vi "1D history all datatypes.vi"   [LabVIEW 2021, in "Ring Buffer Strict Accessor Unit Tests.lvlib"]
uses:
  Ring Buffer Strict Accessor Unit Tests.lvlib
  ffb6f79c-0e8b-4f28-b3ed-bf3963fddc00.vi
  dcb4b22f-e317-4554-9adc-d9d904393cee.vi
  860586e6-507f-4244-af87-8e25528c7787.vi
  04da1d12-4007-43e6-bd40-3bc5b4287603.vi
  d3cdd860-2221-4504-b2d7-d7ebb0f0ee59.vi
  ecb8fbaa-c9af-4774-8849-7f352d3a9ee1.vi
  dba9704d-e78e-47f3-8626-fce484395582.vi
  112621f5-6873-4c6d-a91b-c9d1466c59a4.vi
  7b287e7a-98f1-404d-bc95-c25095b4fc31.vi
  fa233392-5b64-4c8c-836f-c43556db6967.vi
  6d70e3f0-6966-4327-968b-3c5b2aebe7d0.vi
  ffb6f79c-0e8b-4f28-b3ed-bf3963fddc00.vi/8499afdd-f86a-4785-a8f1-e7a09133571a.vi
  ffb6f79c-0e8b-4f28-b3ed-bf3963fddc00.vi/38752bf6-7fea-4fd6-9295-87f253133584.vi
  ffb6f79c-0e8b-4f28-b3ed-bf3963fddc00.vi/d2d864d0-4a0d-406a-953d-2a5df2a8b7c4.vi
  ffb6f79c-0e8b-4f28-b3ed-bf3963fddc00.vi/8f65235b-2f25-4f49-b818-5875480b4ea3.vi
  dcb4b22f-e317-4554-9adc-d9d904393cee.vi/8499afdd-f86a-4785-a8f1-e7a09133571a.vi
  dcb4b22f-e317-4554-9adc-d9d904393cee.vi/38752bf6-7fea-4fd6-9295-87f253133584.vi
  dcb4b22f-e317-4554-9adc-d9d904393cee.vi/d2d864d0-4a0d-406a-953d-2a5df2a8b7c4.vi
  dcb4b22f-e317-4554-9adc-d9d904393cee.vi/8f65235b-2f25-4f49-b818-5875480b4ea3.vi
  860586e6-507f-4244-af87-8e25528c7787.vi/8499afdd-f86a-4785-a8f1-e7a09133571a.vi
  860586e6-507f-4244-af87-8e25528c7787.vi/38752bf6-7fea-4fd6-9295-87f253133584.vi
  860586e6-507f-4244-af87-8e25528c7787.vi/d2d864d0-4a0d-406a-953d-2a5df2a8b7c4.vi
  860586e6-507f-4244-af87-8e25528c7787.vi/8f65235b-2f25-4f49-b818-5875480b4ea3.vi
  04da1d12-4007-43e6-bd40-3bc5b4287603.vi/8499afdd-f86a-4785-a8f1-e7a09133571a.vi
  04da1d12-4007-43e6-bd40-3bc5b4287603.vi/38752bf6-7fea-4fd6-9295-87f253133584.vi
  04da1d12-4007-43e6-bd40-3bc5b4287603.vi/d2d864d0-4a0d-406a-953d-2a5df2a8b7c4.vi
  04da1d12-4007-43e6-bd40-3bc5b4287603.vi/8f65235b-2f25-4f49-b818-5875480b4ea3.vi
  d3cdd860-2221-4504-b2d7-d7ebb0f0ee59.vi/8499afdd-f86a-4785-a8f1-e7a09133571a.vi
  d3cdd860-2221-4504-b2d7-d7ebb0f0ee59.vi/38752bf6-7fea-4fd6-9295-87f253133584.vi
  d3cdd860-2221-4504-b2d7-d7ebb0f0ee59.vi/d2d864d0-4a0d-406a-953d-2a5df2a8b7c4.vi
  d3cdd860-2221-4504-b2d7-d7ebb0f0ee59.vi/8f65235b-2f25-4f49-b818-5875480b4ea3.vi
  ecb8fbaa-c9af-4774-8849-7f352d3a9ee1.vi/8499afdd-f86a-4785-a8f1-e7a09133571a.vi
  ecb8fbaa-c9af-4774-8849-7f352d3a9ee1.vi/38752bf6-7fea-4fd6-9295-87f253133584.vi
  ecb8fbaa-c9af-4774-8849-7f352d3a9ee1.vi/d2d864d0-4a0d-406a-953d-2a5df2a8b7c4.vi
  ecb8fbaa-c9af-4774-8849-7f352d3a9ee1.vi/8f65235b-2f25-4f49-b818-5875480b4ea3.vi
  dba9704d-e78e-47f3-8626-fce484395582.vi/8499afdd-f86a-4785-a8f1-e7a09133571a.vi
  dba9704d-e78e-47f3-8626-fce484395582.vi/38752bf6-7fea-4fd6-9295-87f253133584.vi
  dba9704d-e78e-47f3-8626-fce484395582.vi/d2d864d0-4a0d-406a-953d-2a5df2a8b7c4.vi
  dba9704d-e78e-47f3-8626-fce484395582.vi/8f65235b-2f25-4f49-b818-5875480b4ea3.vi
  112621f5-6873-4c6d-a91b-c9d1466c59a4.vi/8499afdd-f86a-4785-a8f1-e7a09133571a.vi
  112621f5-6873-4c6d-a91b-c9d1466c59a4.vi/38752bf6-7fea-4fd6-9295-87f253133584.vi
  112621f5-6873-4c6d-a91b-c9d1466c59a4.vi/d2d864d0-4a0d-406a-953d-2a5df2a8b7c4.vi
  112621f5-6873-4c6d-a91b-c9d1466c59a4.vi/8f65235b-2f25-4f49-b818-5875480b4ea3.vi
  7b287e7a-98f1-404d-bc95-c25095b4fc31.vi/8499afdd-f86a-4785-a8f1-e7a09133571a.vi
  7b287e7a-98f1-404d-bc95-c25095b4fc31.vi/38752bf6-7fea-4fd6-9295-87f253133584.vi
  7b287e7a-98f1-404d-bc95-c25095b4fc31.vi/d2d864d0-4a0d-406a-953d-2a5df2a8b7c4.vi
  7b287e7a-98f1-404d-bc95-c25095b4fc31.vi/8f65235b-2f25-4f49-b818-5875480b4ea3.vi
  fa233392-5b64-4c8c-836f-c43556db6967.vi/8499afdd-f86a-4785-a8f1-e7a09133571a.vi
  fa233392-5b64-4c8c-836f-c43556db6967.vi/38752bf6-7fea-4fd6-9295-87f253133584.vi
  fa233392-5b64-4c8c-836f-c43556db6967.vi/d2d864d0-4a0d-406a-953d-2a5df2a8b7c4.vi
  fa233392-5b64-4c8c-836f-c43556db6967.vi/8f65235b-2f25-4f49-b818-5875480b4ea3.vi
  6d70e3f0-6966-4327-968b-3c5b2aebe7d0.vi/8499afdd-f86a-4785-a8f1-e7a09133571a.vi
  6d70e3f0-6966-4327-968b-3c5b2aebe7d0.vi/38752bf6-7fea-4fd6-9295-87f253133584.vi
  6d70e3f0-6966-4327-968b-3c5b2aebe7d0.vi/d2d864d0-4a0d-406a-953d-2a5df2a8b7c4.vi
  6d70e3f0-6966-4327-968b-3c5b2aebe7d0.vi/8f65235b-2f25-4f49-b818-5875480b4ea3.vi
  <userlib>/bjustice/Ring Buffer for Time Series Data/API Poly.vi
  <userlib>/bjustice/Ring Buffer for Time Series Data/API/Write Array.vi
  ffb6f79c-0e8b-4f28-b3ed-bf3963fddc00.vi/8499afdd-f86a-4785-a8f1-e7a09133571a.vi/f2df9050-0eef-46c6-aff6-3ce3a8893ea5.vi
  ffb6f79c-0e8b-4f28-b3ed-bf3963fddc00.vi/38752bf6-7fea-4fd6-9295-87f253133584.vi/17d75e1a-130a-47e0-8f2c-6c7d90b8ca77.vi
  <userlib>/bjustice/Ring Buffer for Time Series Data/API/Read Full Rotated Buffer.vi
  Source/SubVIs/Search for time to keep.vi
  Source/SubVIs/Index ByteArray.vi
  ffb6f79c-0e8b-4f28-b3ed-bf3963fddc00.vi/38752bf6-7fea-4fd6-9295-87f253133584.vi/19bdd28a-0674-4be3-87bb-ec701e431d75.vi
  Source/SubVIs/error if empty buffer.vi
  ffb6f79c-0e8b-4f28-b3ed-bf3963fddc00.vi/8f65235b-2f25-4f49-b818-5875480b4ea3.vi/4c2a6c61-f100-483c-8a49-51e57025a24c.vi
  ffb6f79c-0e8b-4f28-b3ed-bf3963fddc00.vi/8f65235b-2f25-4f49-b818-5875480b4ea3.vi/e57bc314-87c7-4952-9bc8-929005dac297.vi
  dcb4b22f-e317-4554-9adc-d9d904393cee.vi/8499afdd-f86a-4785-a8f1-e7a09133571a.vi/f2df9050-0eef-46c6-aff6-3ce3a8893ea5.vi
  dcb4b22f-e317-4554-9adc-d9d904393cee.vi/38752bf6-7fea-4fd6-9295-87f253133584.vi/17d75e1a-130a-47e0-8f2c-6c7d90b8ca77.vi
  dcb4b22f-e317-4554-9adc-d9d904393cee.vi/38752bf6-7fea-4fd6-9295-87f253133584.vi/19bdd28a-0674-4be3-87bb-ec701e431d75.vi
  dcb4b22f-e317-4554-9adc-d9d904393cee.vi/8f65235b-2f25-4f49-b818-5875480b4ea3.vi/4c2a6c61-f100-483c-8a49-51e57025a24c.vi
  dcb4b22f-e317-4554-9adc-d9d904393cee.vi/8f65235b-2f25-4f49-b818-5875480b4ea3.vi/e57bc314-87c7-4952-9bc8-929005dac297.vi
  860586e6-507f-4244-af87-8e25528c7787.vi/8499afdd-f86a-4785-a8f1-e7a09133571a.vi/f2df9050-0eef-46c6-aff6-3ce3a8893ea5.vi
  860586e6-507f-4244-af87-8e25528c7787.vi/38752bf6-7fea-4fd6-9295-87f253133584.vi/17d75e1a-130a-47e0-8f2c-6c7d90b8ca77.vi
  860586e6-507f-4244-af87-8e25528c7787.vi/38752bf6-7fea-4fd6-9295-87f253133584.vi/19bdd28a-0674-4be3-87bb-ec701e431d75.vi
  860586e6-507f-4244-af87-8e25528c7787.vi/8f65235b-2f25-4f49-b818-5875480b4ea3.vi/4c2a6c61-f100-483c-8a49-51e57025a24c.vi
  860586e6-507f-4244-af87-8e25528c7787.vi/8f65235b-2f25-4f49-b818-5875480b4ea3.vi/e57bc314-87c7-4952-9bc8-929005dac297.vi
  04da1d12-4007-43e6-bd40-3bc5b4287603.vi/8499afdd-f86a-4785-a8f1-e7a09133571a.vi/f2df9050-0eef-46c6-aff6-3ce3a8893ea5.vi
  04da1d12-4007-43e6-bd40-3bc5b4287603.vi/38752bf6-7fea-4fd6-9295-87f253133584.vi/17d75e1a-130a-47e0-8f2c-6c7d90b8ca77.vi
  04da1d12-4007-43e6-bd40-3bc5b4287603.vi/38752bf6-7fea-4fd6-9295-87f253133584.vi/19bdd28a-0674-4be3-87bb-ec701e431d75.vi
  04da1d12-4007-43e6-bd40-3bc5b4287603.vi/8f65235b-2f25-4f49-b818-5875480b4ea3.vi/4c2a6c61-f100-483c-8a49-51e57025a24c.vi
  04da1d12-4007-43e6-bd40-3bc5b4287603.vi/8f65235b-2f25-4f49-b818-5875480b4ea3.vi/e57bc314-87c7-4952-9bc8-929005dac297.vi
  d3cdd860-2221-4504-b2d7-d7ebb0f0ee59.vi/8499afdd-f86a-4785-a8f1-e7a09133571a.vi/f2df9050-0eef-46c6-aff6-3ce3a8893ea5.vi
  d3cdd860-2221-4504-b2d7-d7ebb0f0ee59.vi/38752bf6-7fea-4fd6-9295-87f253133584.vi/17d75e1a-130a-47e0-8f2c-6c7d90b8ca77.vi
  d3cdd860-2221-4504-b2d7-d7ebb0f0ee59.vi/38752bf6-7fea-4fd6-9295-87f253133584.vi/19bdd28a-0674-4be3-87bb-ec701e431d75.vi
  d3cdd860-2221-4504-b2d7-d7ebb0f0ee59.vi/8f65235b-2f25-4f49-b818-5875480b4ea3.vi/4c2a6c61-f100-483c-8a49-51e57025a24c.vi
  d3cdd860-2221-4504-b2d7-d7ebb0f0ee59.vi/8f65235b-2f25-4f49-b818-5875480b4ea3.vi/e57bc314-87c7-4952-9bc8-929005dac297.vi
  ecb8fbaa-c9af-4774-8849-7f352d3a9ee1.vi/8499afdd-f86a-4785-a8f1-e7a09133571a.vi/f2df9050-0eef-46c6-aff6-3ce3a8893ea5.vi
  ecb8fbaa-c9af-4774-8849-7f352d3a9ee1.vi/38752bf6-7fea-4fd6-9295-87f253133584.vi/17d75e1a-130a-47e0-8f2c-6c7d90b8ca77.vi
  ecb8fbaa-c9af-4774-8849-7f352d3a9ee1.vi/38752bf6-7fea-4fd6-9295-87f253133584.vi/19bdd28a-0674-4be3-87bb-ec701e431d75.vi
  ecb8fbaa-c9af-4774-8849-7f352d3a9ee1.vi/8f65235b-2f25-4f49-b818-5875480b4ea3.vi/4c2a6c61-f100-483c-8a49-51e57025a24c.vi
  ecb8fbaa-c9af-4774-8849-7f352d3a9ee1.vi/8f65235b-2f25-4f49-b818-5875480b4ea3.vi/e57bc314-87c7-4952-9bc8-929005dac297.vi
  dba9704d-e78e-47f3-8626-fce484395582.vi/8499afdd-f86a-4785-a8f1-e7a09133571a.vi/f2df9050-0eef-46c6-aff6-3ce3a8893ea5.vi
  dba9704d-e78e-47f3-8626-fce484395582.vi/38752bf6-7fea-4fd6-9295-87f253133584.vi/17d75e1a-130a-47e0-8f2c-6c7d90b8ca77.vi
  dba9704d-e78e-47f3-8626-fce484395582.vi/38752bf6-7fea-4fd6-9295-87f253133584.vi/19bdd28a-0674-4be3-87bb-ec701e431d75.vi
  dba9704d-e78e-47f3-8626-fce484395582.vi/8f65235b-2f25-4f49-b818-5875480b4ea3.vi/4c2a6c61-f100-483c-8a49-51e57025a24c.vi
  dba9704d-e78e-47f3-8626-fce484395582.vi/8f65235b-2f25-4f49-b818-5875480b4ea3.vi/e57bc314-87c7-4952-9bc8-929005dac297.vi
  112621f5-6873-4c6d-a91b-c9d1466c59a4.vi/8499afdd-f86a-4785-a8f1-e7a09133571a.vi/f2df9050-0eef-46c6-aff6-3ce3a8893ea5.vi
  112621f5-6873-4c6d-a91b-c9d1466c59a4.vi/38752bf6-7fea-4fd6-9295-87f253133584.vi/17d75e1a-130a-47e0-8f2c-6c7d90b8ca77.vi
  112621f5-6873-4c6d-a91b-c9d1466c59a4.vi/38752bf6-7fea-4fd6-9295-87f253133584.vi/19bdd28a-0674-4be3-87bb-ec701e431d75.vi
  112621f5-6873-4c6d-a91b-c9d1466c59a4.vi/8f65235b-2f25-4f49-b818-5875480b4ea3.vi/4c2a6c61-f100-483c-8a49-51e57025a24c.vi
  112621f5-6873-4c6d-a91b-c9d1466c59a4.vi/8f65235b-2f25-4f49-b818-5875480b4ea3.vi/e57bc314-87c7-4952-9bc8-929005dac297.vi
  7b287e7a-98f1-404d-bc95-c25095b4fc31.vi/8499afdd-f86a-4785-a8f1-e7a09133571a.vi/f2df9050-0eef-46c6-aff6-3ce3a8893ea5.vi
  7b287e7a-98f1-404d-bc95-c25095b4fc31.vi/38752bf6-7fea-4fd6-9295-87f253133584.vi/17d75e1a-130a-47e0-8f2c-6c7d90b8ca77.vi
  7b287e7a-98f1-404d-bc95-c25095b4fc31.vi/38752bf6-7fea-4fd6-9295-87f253133584.vi/19bdd28a-0674-4be3-87bb-ec701e431d75.vi
  7b287e7a-98f1-404d-bc95-c25095b4fc31.vi/8f65235b-2f25-4f49-b818-5875480b4ea3.vi/4c2a6c61-f100-483c-8a49-51e57025a24c.vi
  7b287e7a-98f1-404d-bc95-c25095b4fc31.vi/8f65235b-2f25-4f49-b818-5875480b4ea3.vi/e57bc314-87c7-4952-9bc8-929005dac297.vi
  fa233392-5b64-4c8c-836f-c43556db6967.vi/8499afdd-f86a-4785-a8f1-e7a09133571a.vi/f2df9050-0eef-46c6-aff6-3ce3a8893ea5.vi
  fa233392-5b64-4c8c-836f-c43556db6967.vi/38752bf6-7fea-4fd6-9295-87f253133584.vi/17d75e1a-130a-47e0-8f2c-6c7d90b8ca77.vi
  fa233392-5b64-4c8c-836f-c43556db6967.vi/38752bf6-7fea-4fd6-9295-87f253133584.vi/19bdd28a-0674-4be3-87bb-ec701e431d75.vi
  fa233392-5b64-4c8c-836f-c43556db6967.vi/8f65235b-2f25-4f49-b818-5875480b4ea3.vi/4c2a6c61-f100-483c-8a49-51e57025a24c.vi
  fa233392-5b64-4c8c-836f-c43556db6967.vi/8f65235b-2f25-4f49-b818-5875480b4ea3.vi/e57bc314-87c7-4952-9bc8-929005dac297.vi
  6d70e3f0-6966-4327-968b-3c5b2aebe7d0.vi/8499afdd-f86a-4785-a8f1-e7a09133571a.vi/f2df9050-0eef-46c6-aff6-3ce3a8893ea5.vi
  6d70e3f0-6966-4327-968b-3c5b2aebe7d0.vi/38752bf6-7fea-4fd6-9295-87f253133584.vi/17d75e1a-130a-47e0-8f2c-6c7d90b8ca77.vi
  6d70e3f0-6966-4327-968b-3c5b2aebe7d0.vi/38752bf6-7fea-4fd6-9295-87f253133584.vi/19bdd28a-0674-4be3-87bb-ec701e431d75.vi
  6d70e3f0-6966-4327-968b-3c5b2aebe7d0.vi/8f65235b-2f25-4f49-b818-5875480b4ea3.vi/4c2a6c61-f100-483c-8a49-51e57025a24c.vi
  6d70e3f0-6966-4327-968b-3c5b2aebe7d0.vi/8f65235b-2f25-4f49-b818-5875480b4ea3.vi/e57bc314-87c7-4952-9bc8-929005dac297.vi
  <userlib>/bjustice/Ring Buffer for Time Series Data/SubVIs/Split Values Array.vi
  <userlib>/bjustice/Ring Buffer for Time Series Data/SubVIs/Replace Values Array Multiple Timestamps.vi
  ffb6f79c-0e8b-4f28-b3ed-bf3963fddc00.vi/8499afdd-f86a-4785-a8f1-e7a09133571a.vi/f2df9050-0eef-46c6-aff6-3ce3a8893ea5.vi/63c583a5-c20f-4aba-9c90-661423dee4c4.vi
  ffb6f79c-0e8b-4f28-b3ed-bf3963fddc00.vi/8499afdd-f86a-4785-a8f1-e7a09133571a.vi/f2df9050-0eef-46c6-aff6-3ce3a8893ea5.vi/52385341-3d9c-45d2-aff5-e082a4793eb1.vi
  ffb6f79c-0e8b-4f28-b3ed-bf3963fddc00.vi/8499afdd-f86a-4785-a8f1-e7a09133571a.vi/f2df9050-0eef-46c6-aff6-3ce3a8893ea5.vi/37f29efa-f142-46b1-a185-f0098a95fbb6.vi
  ffb6f79c-0e8b-4f28-b3ed-bf3963fddc00.vi/8499afdd-f86a-4785-a8f1-e7a09133571a.vi/f2df9050-0eef-46c6-aff6-3ce3a8893ea5.vi/84b3d231-9afe-4b6e-afae-e0be43a31e4e.vi
  ffb6f79c-0e8b-4f28-b3ed-bf3963fddc00.vi/8499afdd-f86a-4785-a8f1-e7a09133571a.vi/f2df9050-0eef-46c6-aff6-3ce3a8893ea5.vi/c726271c-fc36-4bb7-8553-8945ec40c1cd.vi
  ffb6f79c-0e8b-4f28-b3ed-bf3963fddc00.vi/8499afdd-f86a-4785-a8f1-e7a09133571a.vi/f2df9050-0eef-46c6-aff6-3ce3a8893ea5.vi/a7b1d944-dc88-46f5-9d3e-305d46bbe1f6.vi
  ffb6f79c-0e8b-4f28-b3ed-bf3963fddc00.vi/8499afdd-f86a-4785-a8f1-e7a09133571a.vi/f2df9050-0eef-46c6-aff6-3ce3a8893ea5.vi/8abc4a6e-a1d2-4e85-879b-517e0ab55733.vi
  ffb6f79c-0e8b-4f28-b3ed-bf3963fddc00.vi/8499afdd-f86a-4785-a8f1-e7a09133571a.vi/f2df9050-0eef-46c6-aff6-3ce3a8893ea5.vi/bd347357-b475-4a03-9ac5-3b85ef11aecc.vi
  ffb6f79c-0e8b-4f28-b3ed-bf3963fddc00.vi/8499afdd-f86a-4785-a8f1-e7a09133571a.vi/f2df9050-0eef-46c6-aff6-3ce3a8893ea5.vi/391b36e9-a702-45e4-9499-3914f8833a58.vi
  ffb6f79c-0e8b-4f28-b3ed-bf3963fddc00.vi/8499afdd-f86a-4785-a8f1-e7a09133571a.vi/f2df9050-0eef-46c6-aff6-3ce3a8893ea5.vi/44155b33-c915-49ce-9e44-a66693aa70dd.vi
  ffb6f79c-0e8b-4f28-b3ed-bf3963fddc00.vi/8499afdd-f86a-4785-a8f1-e7a09133571a.vi/f2df9050-0eef-46c6-aff6-3ce3a8893ea5.vi/36977d53-dbe0-4dbc-b2ac-3dea4345b868.vi
  ffb6f79c-0e8b-4f28-b3ed-bf3963fddc00.vi/38752bf6-7fea-4fd6-9295-87f253133584.vi/17d75e1a-130a-47e0-8f2c-6c7d90b8ca77.vi/bbb64351-fa28-4ac1-b583-44e271193ecd.vi
  <userlib>/bjustice/Ring Buffer for Time Series Data/SubVIs/Rotate Buffer.vi
  Source/SubVIs/Search for oldest time to keep.vi
  Source/SubVIs/Search for newest time to keep.vi
  Source/SubVIs/datatype byte size.vi
  Source/SubVIs/array sizes to number of points.vi
  ffb6f79c-0e8b-4f28-b3ed-bf3963fddc00.vi/38752bf6-7fea-4fd6-9295-87f253133584.vi/19bdd28a-0674-4be3-87bb-ec701e431d75.vi/81c66277-30bd-484c-9c7c-9646f36721bb.vi
  ffb6f79c-0e8b-4f28-b3ed-bf3963fddc00.vi/38752bf6-7fea-4fd6-9295-87f253133584.vi/19bdd28a-0674-4be3-87bb-ec701e431d75.vi/7ca10173-70f1-4bfb-9c4b-948090662032.vi
  ffb6f79c-0e8b-4f28-b3ed-bf3963fddc00.vi/38752bf6-7fea-4fd6-9295-87f253133584.vi/19bdd28a-0674-4be3-87bb-ec701e431d75.vi/ea4aced9-3494-4b3f-b998-02af6afbdac4.vi
  ffb6f79c-0e8b-4f28-b3ed-bf3963fddc00.vi/38752bf6-7fea-4fd6-9295-87f253133584.vi/19bdd28a-0674-4be3-87bb-ec701e431d75.vi/022c581c-5349-49df-98f9-5a038829ee63.vi
  ffb6f79c-0e8b-4f28-b3ed-bf3963fddc00.vi/38752bf6-7fea-4fd6-9295-87f253133584.vi/19bdd28a-0674-4be3-87bb-ec701e431d75.vi/ed40bcc8-bbaa-4b61-9e1a-b4b75cf21b06.vi
  ffb6f79c-0e8b-4f28-b3ed-bf3963fddc00.vi/38752bf6-7fea-4fd6-9295-87f253133584.vi/19bdd28a-0674-4be3-87bb-ec701e431d75.vi/f4b703c2-aaab-40a0-b3da-b0c22dc82d50.vi
  ffb6f79c-0e8b-4f28-b3ed-bf3963fddc00.vi/38752bf6-7fea-4fd6-9295-87f253133584.vi/19bdd28a-0674-4be3-87bb-ec701e431d75.vi/1efa054f-b143-4d96-9f7e-584a7c6fa7fd.vi
  ffb6f79c-0e8b-4f28-b3ed-bf3963fddc00.vi/38752bf6-7fea-4fd6-9295-87f253133584.vi/19bdd28a-0674-4be3-87bb-ec701e431d75.vi/b7c29f3f-256a-4401-af9d-aa15374df391.vi
  ffb6f79c-0e8b-4f28-b3ed-bf3963fddc00.vi/38752bf6-7fea-4fd6-9295-87f253133584.vi/19bdd28a-0674-4be3-87bb-ec701e431d75.vi/2fb7b479-974d-4a18-8674-c4c8d9dc9a89.vi
  ffb6f79c-0e8b-4f28-b3ed-bf3963fddc00.vi/38752bf6-7fea-4fd6-9295-87f253133584.vi/19bdd28a-0674-4be3-87bb-ec701e431d75.vi/faac7175-5814-4bb6-a961-a8db1f460653.vi
  ffb6f79c-0e8b-4f28-b3ed-bf3963fddc00.vi/38752bf6-7fea-4fd6-9295-87f253133584.vi/19bdd28a-0674-4be3-87bb-ec701e431d75.vi/b6af2a6f-71a4-4cfe-837f-b196861458b0.vi
  dcb4b22f-e317-4554-9adc-d9d904393cee.vi/8499afdd-f86a-4785-a8f1-e7a09133571a.vi/f2df9050-0eef-46c6-aff6-3ce3a8893ea5.vi/63c583a5-c20f-4aba-9c90-661423dee4c4.vi
  dcb4b22f-e317-4554-9adc-d9d904393cee.vi/8499afdd-f86a-4785-a8f1-e7a09133571a.vi/f2df9050-0eef-46c6-aff6-3ce3a8893ea5.vi/52385341-3d9c-45d2-aff5-e082a4793eb1.vi
  dcb4b22f-e317-4554-9adc-d9d904393cee.vi/8499afdd-f86a-4785-a8f1-e7a09133571a.vi/f2df9050-0eef-46c6-aff6-3ce3a8893ea5.vi/37f29efa-f142-46b1-a185-f0098a95fbb6.vi
  dcb4b22f-e317-4554-9adc-d9d904393cee.vi/8499afdd-f86a-4785-a8f1-e7a09133571a.vi/f2df9050-0eef-46c6-aff6-3ce3a8893ea5.vi/84b3d231-9afe-4b6e-afae-e0be43a31e4e.vi
  dcb4b22f-e317-4554-9adc-d9d904393cee.vi/8499afdd-f86a-4785-a8f1-e7a09133571a.vi/f2df9050-0eef-46c6-aff6-3ce3a8893ea5.vi/c726271c-fc36-4bb7-8553-8945ec40c1cd.vi
  dcb4b22f-e317-4554-9adc-d9d904393cee.vi/8499afdd-f86a-4785-a8f1-e7a09133571a.vi/f2df9050-0eef-46c6-aff6-3ce3a8893ea5.vi/a7b1d944-dc88-46f5-9d3e-305d46bbe1f6.vi
  dcb4b22f-e317-4554-9adc-d9d904393cee.vi/8499afdd-f86a-4785-a8f1-e7a09133571a.vi/f2df9050-0eef-46c6-aff6-3ce3a8893ea5.vi/8abc4a6e-a1d2-4e85-879b-517e0ab55733.vi
  dcb4b22f-e317-4554-9adc-d9d904393cee.vi/8499afdd-f86a-4785-a8f1-e7a09133571a.vi/f2df9050-0eef-46c6-aff6-3ce3a8893ea5.vi/bd347357-b475-4a03-9ac5-3b85ef11aecc.vi
  dcb4b22f-e317-4554-9adc-d9d904393cee.vi/8499afdd-f86a-4785-a8f1-e7a09133571a.vi/f2df9050-0eef-46c6-aff6-3ce3a8893ea5.vi/391b36e9-a702-45e4-9499-3914f8833a58.vi
  dcb4b22f-e317-4554-9adc-d9d904393cee.vi/8499afdd-f86a-4785-a8f1-e7a09133571a.vi/f2df9050-0eef-46c6-aff6-3ce3a8893ea5.vi/44155b33-c915-49ce-9e44-a66693aa70dd.vi
  dcb4b22f-e317-4554-9adc-d9d904393cee.vi/8499afdd-f86a-4785-a8f1-e7a09133571a.vi/f2df9050-0eef-46c6-aff6-3ce3a8893ea5.vi/36977d53-dbe0-4dbc-b2ac-3dea4345b868.vi
  dcb4b22f-e317-4554-9adc-d9d904393cee.vi/38752bf6-7fea-4fd6-9295-87f253133584.vi/17d75e1a-130a-47e0-8f2c-6c7d90b8ca77.vi/bbb64351-fa28-4ac1-b583-44e271193ecd.vi
  dcb4b22f-e317-4554-9adc-d9d904393cee.vi/38752bf6-7fea-4fd6-9295-87f253133584.vi/19bdd28a-0674-4be3-87bb-ec701e431d75.vi/81c66277-30bd-484c-9c7c-9646f36721bb.vi
  dcb4b22f-e317-4554-9adc-d9d904393cee.vi/38752bf6-7fea-4fd6-9295-87f253133584.vi/19bdd28a-0674-4be3-87bb-ec701e431d75.vi/7ca10173-70f1-4bfb-9c4b-948090662032.vi
  dcb4b22f-e317-4554-9adc-d9d904393cee.vi/38752bf6-7fea-4fd6-9295-87f253133584.vi/19bdd28a-0674-4be3-87bb-ec701e431d75.vi/ea4aced9-3494-4b3f-b998-02af6afbdac4.vi
  dcb4b22f-e317-4554-9adc-d9d904393cee.vi/38752bf6-7fea-4fd6-9295-87f253133584.vi/19bdd28a-0674-4be3-87bb-ec701e431d75.vi/022c581c-5349-49df-98f9-5a038829ee63.vi
  dcb4b22f-e317-4554-9adc-d9d904393cee.vi/38752bf6-7fea-4fd6-9295-87f253133584.vi/19bdd28a-0674-4be3-87bb-ec701e431d75.vi/ed40bcc8-bbaa-4b61-9e1a-b4b75cf21b06.vi
  dcb4b22f-e317-4554-9adc-d9d904393cee.vi/38752bf6-7fea-4fd6-9295-87f253133584.vi/19bdd28a-0674-4be3-87bb-ec701e431d75.vi/f4b703c2-aaab-40a0-b3da-b0c22dc82d50.vi
  dcb4b22f-e317-4554-9adc-d9d904393cee.vi/38752bf6-7fea-4fd6-9295-87f253133584.vi/19bdd28a-0674-4be3-87bb-ec701e431d75.vi/1efa054f-b143-4d96-9f7e-584a7c6fa7fd.vi
  dcb4b22f-e317-4554-9adc-d9d904393cee.vi/38752bf6-7fea-4fd6-9295-87f253133584.vi/19bdd28a-0674-4be3-87bb-ec701e431d75.vi/b7c29f3f-256a-4401-af9d-aa15374df391.vi
  dcb4b22f-e317-4554-9adc-d9d904393cee.vi/38752bf6-7fea-4fd6-9295-87f253133584.vi/19bdd28a-0674-4be3-87bb-ec701e431d75.vi/2fb7b479-974d-4a18-8674-c4c8d9dc9a89.vi
  dcb4b22f-e317-4554-9adc-d9d904393cee.vi/38752bf6-7fea-4fd6-9295-87f253133584.vi/19bdd28a-0674-4be3-87bb-ec701e431d75.vi/faac7175-5814-4bb6-a961-a8db1f460653.vi
  dcb4b22f-e317-4554-9adc-d9d904393cee.vi/38752bf6-7fea-4fd6-9295-87f253133584.vi/19bdd28a-0674-4be3-87bb-ec701e431d75.vi/b6af2a6f-71a4-4cfe-837f-b196861458b0.vi
  860586e6-507f-4244-af87-8e25528c7787.vi/8499afdd-f86a-4785-a8f1-e7a09133571a.vi/f2df9050-0eef-46c6-aff6-3ce3a8893ea5.vi/63c583a5-c20f-4aba-9c90-661423dee4c4.vi
  860586e6-507f-4244-af87-8e25528c7787.vi/8499afdd-f86a-4785-a8f1-e7a09133571a.vi/f2df9050-0eef-46c6-aff6-3ce3a8893ea5.vi/52385341-3d9c-45d2-aff5-e082a4793eb1.vi
  860586e6-507f-4244-af87-8e25528c7787.vi/8499afdd-f86a-4785-a8f1-e7a09133571a.vi/f2df9050-0eef-46c6-aff6-3ce3a8893ea5.vi/37f29efa-f142-46b1-a185-f0098a95fbb6.vi
  860586e6-507f-4244-af87-8e25528c7787.vi/8499afdd-f86a-4785-a8f1-e7a09133571a.vi/f2df9050-0eef-46c6-aff6-3ce3a8893ea5.vi/84b3d231-9afe-4b6e-afae-e0be43a31e4e.vi
  860586e6-507f-4244-af87-8e25528c7787.vi/8499afdd-f86a-4785-a8f1-e7a09133571a.vi/f2df9050-0eef-46c6-aff6-3ce3a8893ea5.vi/c726271c-fc36-4bb7-8553-8945ec40c1cd.vi
  860586e6-507f-4244-af87-8e25528c7787.vi/8499afdd-f86a-4785-a8f1-e7a09133571a.vi/f2df9050-0eef-46c6-aff6-3ce3a8893ea5.vi/a7b1d944-dc88-46f5-9d3e-305d46bbe1f6.vi
  860586e6-507f-4244-af87-8e25528c7787.vi/8499afdd-f86a-4785-a8f1-e7a09133571a.vi/f2df9050-0eef-46c6-aff6-3ce3a8893ea5.vi/8abc4a6e-a1d2-4e85-879b-517e0ab55733.vi
  860586e6-507f-4244-af87-8e25528c7787.vi/8499afdd-f86a-4785-a8f1-e7a09133571a.vi/f2df9050-0eef-46c6-aff6-3ce3a8893ea5.vi/bd347357-b475-4a03-9ac5-3b85ef11aecc.vi
  860586e6-507f-4244-af87-8e25528c7787.vi/8499afdd-f86a-4785-a8f1-e7a09133571a.vi/f2df9050-0eef-46c6-aff6-3ce3a8893ea5.vi/391b36e9-a702-45e4-9499-3914f8833a58.vi
  860586e6-507f-4244-af87-8e25528c7787.vi/8499afdd-f86a-4785-a8f1-e7a09133571a.vi/f2df9050-0eef-46c6-aff6-3ce3a8893ea5.vi/44155b33-c915-49ce-9e44-a66693aa70dd.vi
  860586e6-507f-4244-af87-8e25528c7787.vi/8499afdd-f86a-4785-a8f1-e7a09133571a.vi/f2df9050-0eef-46c6-aff6-3ce3a8893ea5.vi/36977d53-dbe0-4dbc-b2ac-3dea4345b868.vi
  860586e6-507f-4244-af87-8e25528c7787.vi/38752bf6-7fea-4fd6-9295-87f253133584.vi/17d75e1a-130a-47e0-8f2c-6c7d90b8ca77.vi/bbb64351-fa28-4ac1-b583-44e271193ecd.vi
  860586e6-507f-4244-af87-8e25528c7787.vi/38752bf6-7fea-4fd6-9295-87f253133584.vi/19bdd28a-0674-4be3-87bb-ec701e431d75.vi/81c66277-30bd-484c-9c7c-9646f36721bb.vi
  860586e6-507f-4244-af87-8e25528c7787.vi/38752bf6-7fea-4fd6-9295-87f253133584.vi/19bdd28a-0674-4be3-87bb-ec701e431d75.vi/7ca10173-70f1-4bfb-9c4b-948090662032.vi
  860586e6-507f-4244-af87-8e25528c7787.vi/38752bf6-7fea-4fd6-9295-87f253133584.vi/19bdd28a-0674-4be3-87bb-ec701e431d75.vi/ea4aced9-3494-4b3f-b998-02af6afbdac4.vi
  860586e6-507f-4244-af87-8e25528c7787.vi/38752bf6-7fea-4fd6-9295-87f253133584.vi/19bdd28a-0674-4be3-87bb-ec701e431d75.vi/022c581c-5349-49df-98f9-5a038829ee63.vi
  860586e6-507f-4244-af87-8e25528c7787.vi/38752bf6-7fea-4fd6-9295-87f253133584.vi/19bdd28a-0674-4be3-87bb-ec701e431d75.vi/ed40bcc8-bbaa-4b61-9e1a-b4b75cf21b06.vi
  860586e6-507f-4244-af87-8e25528c7787.vi/38752bf6-7fea-4fd6-9295-87f253133584.vi/19bdd28a-0674-4be3-87bb-ec701e431d75.vi/f4b703c2-aaab-40a0-b3da-b0c22dc82d50.vi
  860586e6-507f-4244-af87-8e25528c7787.vi/38752bf6-7fea-4fd6-9295-87f253133584.vi/19bdd28a-0674-4be3-87bb-ec701e431d75.vi/1efa054f-b143-4d96-9f7e-584a7c6fa7fd.vi
  860586e6-507f-4244-af87-8e25528c7787.vi/38752bf6-7fea-4fd6-9295-87f253133584.vi/19bdd28a-0674-4be3-87bb-ec701e431d75.vi/b7c29f3f-256a-4401-af9d-aa15374df391.vi
  860586e6-507f-4244-af87-8e25528c7787.vi/38752bf6-7fea-4fd6-9295-87f253133584.vi/19bdd28a-0674-4be3-87bb-ec701e431d75.vi/2fb7b479-974d-4a18-8674-c4c8d9dc9a89.vi
  860586e6-507f-4244-af87-8e25528c7787.vi/38752bf6-7fea-4fd6-9295-87f253133584.vi/19bdd28a-0674-4be3-87bb-ec701e431d75.vi/faac7175-5814-4bb6-a961-a8db1f460653.vi
  860586e6-507f-4244-af87-8e25528c7787.vi/38752bf6-7fea-4fd6-9295-87f253133584.vi/19bdd28a-0674-4be3-87bb-ec701e431d75.vi/b6af2a6f-71a4-4cfe-837f-b196861458b0.vi
  04da1d12-4007-43e6-bd40-3bc5b4287603.vi/8499afdd-f86a-4785-a8f1-e7a09133571a.vi/f2df9050-0eef-46c6-aff6-3ce3a8893ea5.vi/63c583a5-c20f-4aba-9c90-661423dee4c4.vi
  04da1d12-4007-43e6-bd40-3bc5b4287603.vi/8499afdd-f86a-4785-a8f1-e7a09133571a.vi/f2df9050-0eef-46c6-aff6-3ce3a8893ea5.vi/52385341-3d9c-45d2-aff5-e082a4793eb1.vi
  04da1d12-4007-43e6-bd40-3bc5b4287603.vi/8499afdd-f86a-4785-a8f1-e7a09133571a.vi/f2df9050-0eef-46c6-aff6-3ce3a8893ea5.vi/37f29efa-f142-46b1-a185-f0098a95fbb6.vi
  04da1d12-4007-43e6-bd40-3bc5b4287603.vi/8499afdd-f86a-4785-a8f1-e7a09133571a.vi/f2df9050-0eef-46c6-aff6-3ce3a8893ea5.vi/84b3d231-9afe-4b6e-afae-e0be43a31e4e.vi
  04da1d12-4007-43e6-bd40-3bc5b4287603.vi/8499afdd-f86a-4785-a8f1-e7a09133571a.vi/f2df9050-0eef-46c6-aff6-3ce3a8893ea5.vi/c726271c-fc36-4bb7-8553-8945ec40c1cd.vi
  04da1d12-4007-43e6-bd40-3bc5b4287603.vi/8499afdd-f86a-4785-a8f1-e7a09133571a.vi/f2df9050-0eef-46c6-aff6-3ce3a8893ea5.vi/a7b1d944-dc88-46f5-9d3e-305d46bbe1f6.vi
  04da1d12-4007-43e6-bd40-3bc5b4287603.vi/8499afdd-f86a-4785-a8f1-e7a09133571a.vi/f2df9050-0eef-46c6-aff6-3ce3a8893ea5.vi/8abc4a6e-a1d2-4e85-879b-517e0ab55733.vi
  04da1d12-4007-43e6-bd40-3bc5b4287603.vi/8499afdd-f86a-4785-a8f1-e7a09133571a.vi/f2df9050-0eef-46c6-aff6-3ce3a8893ea5.vi/bd347357-b475-4a03-9ac5-3b85ef11aecc.vi
  04da1d12-4007-43e6-bd40-3bc5b4287603.vi/8499afdd-f86a-4785-a8f1-e7a09133571a.vi/f2df9050-0eef-46c6-aff6-3ce3a8893ea5.vi/391b36e9-a702-45e4-9499-3914f8833a58.vi
  04da1d12-4007-43e6-bd40-3bc5b4287603.vi/8499afdd-f86a-4785-a8f1-e7a09133571a.vi/f2df9050-0eef-46c6-aff6-3ce3a8893ea5.vi/44155b33-c915-49ce-9e44-a66693aa70dd.vi
  04da1d12-4007-43e6-bd40-3bc5b4287603.vi/8499afdd-f86a-4785-a8f1-e7a09133571a.vi/f2df9050-0eef-46c6-aff6-3ce3a8893ea5.vi/36977d53-dbe0-4dbc-b2ac-3dea4345b868.vi
  04da1d12-4007-43e6-bd40-3bc5b4287603.vi/38752bf6-7fea-4fd6-9295-87f253133584.vi/17d75e1a-130a-47e0-8f2c-6c7d90b8ca77.vi/bbb64351-fa28-4ac1-b583-44e271193ecd.vi
  04da1d12-4007-43e6-bd40-3bc5b4287603.vi/38752bf6-7fea-4fd6-9295-87f253133584.vi/19bdd28a-0674-4be3-87bb-ec701e431d75.vi/81c66277-30bd-484c-9c7c-9646f36721bb.vi
  04da1d12-4007-43e6-bd40-3bc5b4287603.vi/38752bf6-7fea-4fd6-9295-87f253133584.vi/19bdd28a-0674-4be3-87bb-ec701e431d75.vi/7ca10173-70f1-4bfb-9c4b-948090662032.vi
  04da1d12-4007-43e6-bd40-3bc5b4287603.vi/38752bf6-7fea-4fd6-9295-87f253133584.vi/19bdd28a-0674-4be3-87bb-ec701e431d75.vi/ea4aced9-3494-4b3f-b998-02af6afbdac4.vi
  04da1d12-4007-43e6-bd40-3bc5b4287603.vi/38752bf6-7fea-4fd6-9295-87f253133584.vi/19bdd28a-0674-4be3-87bb-ec701e431d75.vi/022c581c-5349-49df-98f9-5a038829ee63.vi
  04da1d12-4007-43e6-bd40-3bc5b4287603.vi/38752bf6-7fea-4fd6-9295-87f253133584.vi/19bdd28a-0674-4be3-87bb-ec701e431d75.vi/ed40bcc8-bbaa-4b61-9e1a-b4b75cf21b06.vi
  04da1d12-4007-43e6-bd40-3bc5b4287603.vi/38752bf6-7fea-4fd6-9295-87f253133584.vi/19bdd28a-0674-4be3-87bb-ec701e431d75.vi/f4b703c2-aaab-40a0-b3da-b0c22dc82d50.vi
  04da1d12-4007-43e6-bd40-3bc5b4287603.vi/38752bf6-7fea-4fd6-9295-87f253133584.vi/19bdd28a-0674-4be3-87bb-ec701e431d75.vi/1efa054f-b143-4d96-9f7e-584a7c6fa7fd.vi
  04da1d12-4007-43e6-bd40-3bc5b4287603.vi/38752bf6-7fea-4fd6-9295-87f253133584.vi/19bdd28a-0674-4be3-87bb-ec701e431d75.vi/b7c29f3f-256a-4401-af9d-aa15374df391.vi
  04da1d12-4007-43e6-bd40-3bc5b4287603.vi/38752bf6-7fea-4fd6-9295-87f253133584.vi/19bdd28a-0674-4be3-87bb-ec701e431d75.vi/2fb7b479-974d-4a18-8674-c4c8d9dc9a89.vi
  04da1d12-4007-43e6-bd40-3bc5b4287603.vi/38752bf6-7fea-4fd6-9295-87f253133584.vi/19bdd28a-0674-4be3-87bb-ec701e431d75.vi/faac7175-5814-4bb6-a961-a8db1f460653.vi
  04da1d12-4007-43e6-bd40-3bc5b4287603.vi/38752bf6-7fea-4fd6-9295-87f253133584.vi/19bdd28a-0674-4be3-87bb-ec701e431d75.vi/b6af2a6f-71a4-4cfe-837f-b196861458b0.vi
  d3cdd860-2221-4504-b2d7-d7ebb0f0ee59.vi/8499afdd-f86a-4785-a8f1-e7a09133571a.vi/f2df9050-0eef-46c6-aff6-3ce3a8893ea5.vi/63c583a5-c20f-4aba-9c90-661423dee4c4.vi
  d3cdd860-2221-4504-b2d7-d7ebb0f0ee59.vi/8499afdd-f86a-4785-a8f1-e7a09133571a.vi/f2df9050-0eef-46c6-aff6-3ce3a8893ea5.vi/52385341-3d9c-45d2-aff5-e082a4793eb1.vi
  d3cdd860-2221-4504-b2d7-d7ebb0f0ee59.vi/8499afdd-f86a-4785-a8f1-e7a09133571a.vi/f2df9050-0eef-46c6-aff6-3ce3a8893ea5.vi/37f29efa-f142-46b1-a185-f0098a95fbb6.vi
  d3cdd860-2221-4504-b2d7-d7ebb0f0ee59.vi/8499afdd-f86a-4785-a8f1-e7a09133571a.vi/f2df9050-0eef-46c6-aff6-3ce3a8893ea5.vi/84b3d231-9afe-4b6e-afae-e0be43a31e4e.vi
  d3cdd860-2221-4504-b2d7-d7ebb0f0ee59.vi/8499afdd-f86a-4785-a8f1-e7a09133571a.vi/f2df9050-0eef-46c6-aff6-3ce3a8893ea5.vi/c726271c-fc36-4bb7-8553-8945ec40c1cd.vi
  d3cdd860-2221-4504-b2d7-d7ebb0f0ee59.vi/8499afdd-f86a-4785-a8f1-e7a09133571a.vi/f2df9050-0eef-46c6-aff6-3ce3a8893ea5.vi/a7b1d944-dc88-46f5-9d3e-305d46bbe1f6.vi
  d3cdd860-2221-4504-b2d7-d7ebb0f0ee59.vi/8499afdd-f86a-4785-a8f1-e7a09133571a.vi/f2df9050-0eef-46c6-aff6-3ce3a8893ea5.vi/8abc4a6e-a1d2-4e85-879b-517e0ab55733.vi
  d3cdd860-2221-4504-b2d7-d7ebb0f0ee59.vi/8499afdd-f86a-4785-a8f1-e7a09133571a.vi/f2df9050-0eef-46c6-aff6-3ce3a8893ea5.vi/bd347357-b475-4a03-9ac5-3b85ef11aecc.vi
  d3cdd860-2221-4504-b2d7-d7ebb0f0ee59.vi/8499afdd-f86a-4785-a8f1-e7a09133571a.vi/f2df9050-0eef-46c6-aff6-3ce3a8893ea5.vi/391b36e9-a702-45e4-9499-3914f8833a58.vi
  d3cdd860-2221-4504-b2d7-d7ebb0f0ee59.vi/8499afdd-f86a-4785-a8f1-e7a09133571a.vi/f2df9050-0eef-46c6-aff6-3ce3a8893ea5.vi/44155b33-c915-49ce-9e44-a66693aa70dd.vi
  d3cdd860-2221-4504-b2d7-d7ebb0f0ee59.vi/8499afdd-f86a-4785-a8f1-e7a09133571a.vi/f2df9050-0eef-46c6-aff6-3ce3a8893ea5.vi/36977d53-dbe0-4dbc-b2ac-3dea4345b868.vi
  d3cdd860-2221-4504-b2d7-d7ebb0f0ee59.vi/38752bf6-7fea-4fd6-9295-87f253133584.vi/17d75e1a-130a-47e0-8f2c-6c7d90b8ca77.vi/bbb64351-fa28-4ac1-b583-44e271193ecd.vi
  d3cdd860-2221-4504-b2d7-d7ebb0f0ee59.vi/38752bf6-7fea-4fd6-9295-87f253133584.vi/19bdd28a-0674-4be3-87bb-ec701e431d75.vi/81c66277-30bd-484c-9c7c-9646f36721bb.vi
  d3cdd860-2221-4504-b2d7-d7ebb0f0ee59.vi/38752bf6-7fea-4fd6-9295-87f253133584.vi/19bdd28a-0674-4be3-87bb-ec701e431d75.vi/7ca10173-70f1-4bfb-9c4b-948090662032.vi
  d3cdd860-2221-4504-b2d7-d7ebb0f0ee59.vi/38752bf6-7fea-4fd6-9295-87f253133584.vi/19bdd28a-0674-4be3-87bb-ec701e431d75.vi/ea4aced9-3494-4b3f-b998-02af6afbdac4.vi
  d3cdd860-2221-4504-b2d7-d7ebb0f0ee59.vi/38752bf6-7fea-4fd6-9295-87f253133584.vi/19bdd28a-0674-4be3-87bb-ec701e431d75.vi/022c581c-5349-49df-98f9-5a038829ee63.vi
  d3cdd860-2221-4504-b2d7-d7ebb0f0ee59.vi/38752bf6-7fea-4fd6-9295-87f253133584.vi/19bdd28a-0674-4be3-87bb-ec701e431d75.vi/ed40bcc8-bbaa-4b61-9e1a-b4b75cf21b06.vi
  d3cdd860-2221-4504-b2d7-d7ebb0f0ee59.vi/38752bf6-7fea-4fd6-9295-87f253133584.vi/19bdd28a-0674-4be3-87bb-ec701e431d75.vi/f4b703c2-aaab-40a0-b3da-b0c22dc82d50.vi
  d3cdd860-2221-4504-b2d7-d7ebb0f0ee59.vi/38752bf6-7fea-4fd6-9295-87f253133584.vi/19bdd28a-0674-4be3-87bb-ec701e431d75.vi/1efa054f-b143-4d96-9f7e-584a7c6fa7fd.vi
  d3cdd860-2221-4504-b2d7-d7ebb0f0ee59.vi/38752bf6-7fea-4fd6-9295-87f253133584.vi/19bdd28a-0674-4be3-87bb-ec701e431d75.vi/b7c29f3f-256a-4401-af9d-aa15374df391.vi